vi "UHR-Fleezers Control (host) - 10.2.vi"() -> ()   [LabVIEW 2009] (continued)
  out "All Signals":waveform(dbl)[](graph)=[{"t0"=timestamp(9589.800000000116 s since 1904-01-01), "dt"=0.15, "Y"=[380.0, 400.0], "attributes"=variant("NI_ChannelName"=variant(string "APD 1"))}, {"t0"=timestamp(9589.800000000116 s since 1904-01-01), "dt"=0.15, "Y"=[140.0, 160.0], "attributes"=variant("NI_ChannelName"=variant(string "APD 2"))}, {"t0"=timestamp(9589.800000000116 s since 1904-01-01), "dt"=0.15, "Y"=[-0.5560947071135384, -0.5488051268739088], "attributes"=variant("NI_ChannelName"=variant(string "T1 Y"))}, {"t0"=timestamp(9589.800000000116 s since 1904-01-01), "dt"=0.15, "Y"=[-0.6964523017525798, -0.7003016638635213], "attributes"=variant("NI_ChannelName"=variant(string "T1 X"))}, {"t0"=timestamp(9589.800000000116 s since 1904-01-01), "dt"=0.15, "Y"=[0.009100131229590747, 0.009068117313150425], "attributes"=variant("NI_ChannelName"=variant(string "T1 Sum"))}, {"t0"=timestamp(9589.800000000116 s since 1904-01-01), "dt"=0.15, "Y"=[-0.557341526703397, -0.5498308802934172], "attributes"=variant("NI_ChannelName"=variant(string "T2 Y"))}, {"t0"=timestamp(9589.800000000116 s since 1904-01-01), "dt"=0.15, "Y"=[-0.6977537048097585, -0.7016458986193993], "attributes"=variant("NI_ChannelName"=variant(string "T2 X"))}, {"t0"=timestamp(9589.800000000116 s since 1904-01-01), "dt"=0.15, "Y"=[0.009161107211523788, 0.00913434247871334], "attributes"=variant("NI_ChannelName"=variant(string "T2 Sum"))}, {"t0"=timestamp(9589.800000000116 s since 1904-01-01), "dt"=0.15, "Y"=[0.05199389581726632, 0.0511983167557167], "attributes"=variant("NI_ChannelName"=variant(string "T1 FB X"))}, {"t0"=timestamp(9589.800000000116 s since 1904-01-01), "dt"=0.15, "Y"=[0.016877803888058106, 0.01688229010895108], "attributes"=variant("NI_ChannelName"=variant(string "T1 FB Sum"))}, {"t0"=timestamp(9589.800000000116 s since 1904-01-01), "dt"=0.15, "Y"=[0.048074905987419425, 0.04747925277569201], "attributes"=variant("NI_ChannelName"=variant(string "T2 FB X"))}, {"t0"=timestamp(9589.800000000116 s since 1904-01-01), "dt"=0.15, "Y"=[0.016815240943632313, 0.016807855464339123], "attributes"=variant("NI_ChannelName"=variant(string "T2 FB Sum"))}, {"t0"=timestamp(9589.800000000116 s since 1904-01-01), "dt"=0.15, "Y"=[-3.8792427407756658, -3.877178718972479], "attributes"=variant("NI_ChannelName"=variant(string "PSD Y"))}, {"t0"=timestamp(9589.800000000116 s since 1904-01-01), "dt"=0.15, "Y"=[-0.32047881103365267, -0.32100188649167594], "attributes"=variant("NI_ChannelName"=variant(string "PSD X"))}, {"t0"=timestamp(9589.800000000116 s since 1904-01-01), "dt"=0.15, "Y"=[-0.025290139469588305, -0.02530741294595172], "attributes"=variant("NI_ChannelName"=variant(string "PSD Y Sum"))}]
  in  "Signals to Plot":i32(listbox)
  out "Trap Disp. Freq. (Hz)":dbl=6.666666666666667 caption="Freq. (Hz)" format="%#_6p"
  out "Display Period (s)":dbl=0.15 caption="Period (s)" format="%#_6p"
  in  "Trap Disp. Downsample":dbl=10000.0 caption="Downsample" max=20000.0
  in  "APD Disp. Scale":dbl=0.1 caption="Scale (Divide,\nfor above plot only)"
  in  "APD Disp. Downsample":dbl=15.0 caption="Integrate" min=1.0 max=30.0 step=1.0
  out "APD Display Freq. (Hz)":dbl=6.666666666666667 caption="Freq. (Hz)"
  out "APD Display Period (s)":dbl=0.15 caption="Period (s)"
  out "FFT 1":cluster{"f0":dbl, "df":dbl, "magnitude":dbl[]}[](graph)=[{"f0"=0.0, "df"=3.3333333333333335, "magnitude"=array[10000 elements]}, {"f0"=0.0, "df"=3.3333333333333335, "magnitude"=array[10000 elements]}]
  out "FFT 2":cluster{"f0":dbl, "df":dbl, "magnitude":dbl[]}[](graph)
  in  "FFT 1 Choice 1":u16(ring) items=["T1 Y", "T1 X", "T1 Sum", "T2 Y", "T2 X", "T2 Sum", "T1 FB X", "T1 FB Sum", "T2 FB X", "T2 FB Sum", "PSD Y", "PSD X", "PSD Y Sum", "none"]
  in  "FFT 2 Choice 1":u16(ring)=13 items=["T1 Y", "T1 X", "T1 Sum", "T2 Y", "T2 X", "T2 Sum", "T1 FB X", "T1 FB Sum", "T2 FB X", "T2 FB Sum", "PSD Y", "PSD X", "PSD Y Sum", "none"]
  in  "FFT 1 Choice 2":u16(ring)=1 items=["T1 Y", "T1 X", "T1 Sum", "T2 Y", "T2 X", "T2 Sum", "T1 FB X", "T1 FB Sum", "T2 FB X", "T2 FB Sum", "PSD Y", "PSD X", "PSD Y Sum", "none"]
  in  "FFT 2 Choice 2":u16(ring)=13 items=["T1 Y", "T1 X", "T1 Sum", "T2 Y", "T2 X", "T2 Sum", "T1 FB X", "T1 FB Sum", "T2 FB X", "T2 FB Sum", "PSD Y", "PSD X", "PSD Y Sum", "none"]
  in  "Compute FFT":bool
  in  "Reset FFT":bool
  in  "# Spectra to Ave.":dbl=25.0
  out "Ave. Time (s)":dbl=7.5
  out "1 Channel":waveform(dbl)(graph)={"t0"=timestamp(0 s since 1904-01-01), "dt"=1.4999999999999999e-05, "Y"=array[20000 elements], "attributes"=variant("NI_ChannelName"=variant(string "T1 Y"))}
  out "Slow mean":dbl=0.04741485510254009 format="%0.2f"
  in  "Slow mean N ave.":dbl=1.0 min=1.0 step=1.0
  out "Mean Intensity":dbl=0.04741485510254009
  out "Sigma":dbl=0.006116447585273888
  out "Sigma/Mean":dbl=0.12899855060289364
  in  "Subtract mean":bool
  in  "High Res. Display":u16(ring) items=["T1 Y", "T1 X", "T1 Sum", "T2 Y", "T2 X", "T2 Sum", "T1 FB X", "T1 FB Sum", "T2 FB X", "T2 FB Sum", "PSD Y", "PSD X", "PSD Y Sum"]
  out "APD 1 Rate (Hz)":dbl=330.0 format="%#_3p"
  in  "Tab Control":T4(tab)=enum."APD Counting"
  out "Stage Moving":bool
  in  "Read Cal":bool
  in  "Confocal Linescan":bool
  in  "Speed (nm/s)":dbl=100.0
  in  "Furthest Withdraw (MHz)":dbl=15.0
  in  "Confocal Image":bool
  in  "Round T1 X":bool caption="Round"
  in  "T1 offset_x (mV)":dbl=-63.86439785165793 format="%#_2g"
  in  "T1 kappa_x (pN/nm)":dbl=0.25444062839906995 min=0.0 step=0.001 format="%#_2g"
  out "Time (s)":dbl=8.7
  out "Total Time (s)":dbl=60.0
  in  "Start Saving":bool
  in  "Cal sets to save":u32=50 min=1 step=1
  in  "Comment (data description)":string="testing confocal setup"
  out "Calibrating Trap...":bool
  in  "Trap 2 (ON/OFF)":bool
  in  "Trap 1 (ON/OFF)":bool
  in  "Save Calibration":bool
  in  "N sets to save":u32=200 caption="N Sets"
  in  "Save N Sets":bool
  out "Save file name":path=path "E:/Data/101209/101209_067.dat"
  in  "Save ave N":dbl=500.0 caption="Averaging Factor"
  out "Saving...":bool
  in  "Stop Saving":bool
  out "Progress":u16(slide) scale=0.0..100.0
  out "Manipulating Trap":bool
  out "Buffer Status":dbl(slide) scale=0.0..1.0
  out "Overflow (data lost)":bool
  in  "Reset":bool
  out "Data Rate (Hz)":dbl=66666.66666666667 caption="Trap Data Rate (Hz)" format="%#_3p"
  out "Data Period (s)":dbl=1.4999999999999999e-05 caption="Trap Data Period (s)" format="%#_6p"
  out "Save Data Rate (Hz)":dbl=133.33333333333334 caption="Rate (Hz)" format="%#_6p"
  out "Save Data Period (s)":dbl=0.0075 caption="Period (s)" format="%#_6p"
  in  "T1 alpha_x (nm/V)":dbl=668.456221254379 step=10.0 format="%#_3g"
  in  "T2 alpha_x (nm/V)":dbl=772.4433031277968 step=10.0 format="%#_3g"
  in  "T2 kappa_x (pN/nm)":dbl=0.21976131273941338 min=0.0 step=0.001 format="%#_2g"
  in  "T2 offset_x (mV)":dbl=-64.70019248344109 format="%#_2g"
  in  "BD 1 Frequency 1 (MHz)":dbl=72.0 caption="T1 X (MHz)" min=60.0 max=90.0 step=1.0 format="%#_6p"
  in  "BD 1 Frequency 2 (MHz)":dbl=85.0 caption="T2 X (MHz)" min=60.0 max=90.0 step=1.0 format="%#_6p"
  in  "Green Laser ON/Interlacing":bool
  in  "Round T2 X":bool caption="Round"
  in  "AO1":dbl(slide)=5.724448901115672 caption="Confocal Y (V)" min=0.0 max=10.0 step=0.01 scale=0.0..10.0 scale format="%_1f"
  in  "AO2":dbl(slide)=2.676722922452468 caption="Confocal X (V)" min=0.0 max=10.0 step=0.01 scale=0.0..10.0 scale format="%_1f"
  in  "Trap Raster Scan":bool
  out "Raster Scanning...":bool
  in  "Trap Delta (MHz)":dbl=13.0
  in  "Setpoints (V)":cluster{"Set 1":dbl, "Set 2":dbl}={"Set 1"=9.0, "Set 2"=9.0}
  in  "Index":dbl=67.0 caption="Save File Index" min=1.0 step=1.0
  in  "Position Label 5":string="upper flow spot (UvrD)" caption="5"
  in  "Move to Position":bool
  in  "Position":dbl=1.0 min=1.0 max=10.0 step=1.0
  in  "Set Position":bool
  in  "Saved Stage Positions":dbl[][](array[numeric])=[[1.0, 1.95922, -0.44604, 0.0063], [2.0, 0.0, 0.0, 0.0], [3.0, 2.85199, -0.5102, 0.0063], [4.0, -0.33267, -0.41387, -0.00044], [5.0, 2.804, -1.87124, -0.00044], [6.0, 0.0, 0.0, 0.0], [7.0, 0.0, 0.0, 0.0], [8.0, 0.0, 0.0, 0.0], [9.0, 0.0, 0.0, 0.0], [10.0, 0.0, 0.0, 0.0]]
  in  "Move to Position 5":bool
  in  "z nudge increment (um)":dbl=0.5
  in  "+z":bool
  in  "Position 1 Label":string="Right capillary (DNA beads)" caption="1"
  in  "Set Position 1":bool
  in  "Set Position 2":bool
  in  "Set Position 3":bool
  in  "Set Position 4":bool
  in  "Move to Position 3":bool
  in  "Move to Position 4":bool
  in  "Move to Position 2":bool
  in  "Move to Position 1":bool
  in  "Position 2 Label":string="Left capillary (ADig beads)" caption="2"
  in  "Position 3 Label":string="lower flow spot (ATP)" caption="3"
  in  "Position 4 Label":string="Dump beads" caption="4"
  in  "-z":bool
  in  "Set Position 5":bool
  out "Stage Control Serial Error":errorcluster={"status"=FALSE, "code"=1073676293, "source"="VISA Read in Set Stage Position.vi->UHR-Fleezers Control (host) - 10.2.vi"}
  out "Pump 3 cont disp":string="Left: ADig beads"
  out "Pump 1 cont disp":string="Right: DNA beads "
  in  "Ch 1 Inject Rate (ul/h)":dbl=100.0
  in  "Pump write delay (ms)":dbl=300.0
  in  "All Pump Parameters":T5={"Pump 1"={"Diameter (mm)"=4.61, "Units"=4.0, "Volume"=100.0, "Rate"=100.0}, "Pump 2"={"Diameter (mm)"=4.61, "Units"=3.0, "Volume"=0.0, "Rate"=0.0}, "Pump 3"={"Diameter (mm)"=4.61, "Units"=4.0, "Volume"=100.0, "Rate"=200.0}}
  in  "Ch 2 Inject Volume (uL)":dbl=100.0
  in  "Pump pause delay (ms)":u32
  in  "Ch 3 Inject Volume (uL)":dbl=100.0
  in  "Ch 3 Inject Rate (ul/h)":dbl=200.0
  in  "Flush Center Ch Volume (uL)":dbl=15.0
  in  "Flush Center Ch Rate (ul/m)":dbl=100.0
  in  "Inject Pump 2":bool caption="Inject Pump 2\n(Flush Center)"
  in  "Total Volume\nFlushed (uL)":dbl
  in  "Tab Control 2":T6(tab)=enum."Feedback on Trap Position"
  out "Total Counts (ticks)":u32=600
  in  "Trap ON/OFF X or Y Amp?":bool=TRUE
  in  "Oscillate Set 1":bool
  in  "Trap 1 ON":bool
  in  "Number Interlace Sets":u8=3 min=1 max=3
  in  "DIO count 3 (ticks)":u32=200
  in  "DIO count 2 (ticks)":u32=200
  in  "DIO count 1 (ticks)":u32=200
  in  "BD 2 Amplitude 3 (%)":dbl min=0.0 max=50.0 step=1.0
  in  "BD 2 Amplitude 2 (%)":dbl min=0.0 max=50.0 step=1.0
  in  "BD 2 Amplitude 1 (%)":dbl min=0.0 max=50.0 step=1.0
  in  "BD 1 Amplitude 3 (%)":dbl min=0.0 max=50.0 step=1.0
  in  "BD 1 Amplitude 2 (%)":dbl=35.0 min=0.0 max=50.0 step=1.0
  in  "BD 1 Amplitude 1 (%)":dbl=10.0 min=0.0 max=50.0 step=1.0
  in  "BD 2 Frequency 3 (MHz)":dbl=26.0 min=0.0 max=40.0 step=1.0 format="%#_6p"
  in  "BD 1 Frequency 3 (MHz)":dbl=70.0 min=60.0 max=90.0 step=1.0 format="%#_6p"
  in  "BD 2 Frequency 2 (MHz)":dbl=26.0 min=0.0 max=40.0 step=1.0 format="%#_6p"
  in  "BD 2 Frequency 1 (MHz)":dbl=26.0 min=0.0 max=40.0 step=1.0 format="%#_6p"
  in  "Not-Interlacing Set":enum32{"Set 1", "Set 2", "Set 3"}(radio)
  in  "Interlace":bool=TRUE
  in  "Trap 2 ON":bool
  in  "Trap 3 ON":bool
  in  "Scan axis 2":bool=TRUE
  in  "Osc. freq. (Hz)":dbl=0.25
  in  "Osc. amp. (MHz)":dbl=2.0
  out "Coords":T7
  in  "Manipulation Scaling":cluster{"Horizontal":dbl, "Vertical":dbl}={"Horizontal"=0.075, "Vertical"=0.01}
  in  "Freq or Amp switch first":bool=TRUE
  in  "Swap F1 and F2":bool
  in  "Freq switch delay":u16
  in  "Amp switch delay":u16=5
  in  "MCL Step Increment (V_int)":dbl=3.0
  out "Time to Finish All (min)":dbl=0.13986 format="%#_2p"
  in  "Scan Speed (nm/s)":dbl=100.0
  in  "Scan Range (nm)":dbl=420.0
  in  "Step Size (nm)":dbl=1.0
  in  "MCL/AOM Scale Tweak":dbl=1.0
  in  "MCL Step Position Ratio":dbl=0.5
  in  "Move MCL Also?":bool=TRUE
  out "Final sep (nm)":dbl=1194.000000000001
  out "Initial sep (nm)":dbl=774.0
  out "Save index":dbl=67.0
  out "Final delta (MHz)":dbl=16.41463414634147
  out "Initial delta (MHz)":dbl=13.0
  out "Final freq. (MHz)":dbl=68.58536585365853
  out "Initial freq. (MHz)":dbl=72.0
  in  "Saved AOD Raster Scan Parameter Sets":T8(array[cluster])=[{"Scan Range AOD (nm) 2"=500.0, "Step Size AOD (nm) 2"=1.0, "Scan Speed AOD (nm/s) 2"=100.0, "Number of scans (AOD) 2"=1, "Label"="offset curve"}, {"Scan Range AOD (nm) 2"=420.0, "Step Size AOD (nm) 2"=1.0, "Scan Speed AOD (nm/s) 2"=100.0, "Number of scans (AOD) 2"=1, "Label"="hp raster check"}, {"Scan Range AOD (nm) 2"=6.8, "Step Size AOD (nm) 2"=0.34, "Scan Speed AOD (nm/s) 2"=0.34, "Number of scans (AOD) 2"=1, "Label"="3.4 kbp - 1 bp steps"}]
  in  "Load parameters":bool
  out "Scan Range (MHz)":dbl=-3.4146341463414633
  in  "Restart DMA? (AOD)":bool=TRUE caption="Restart DMA?"
  out "Incr. int (AOD)":i64=-7759651845
  out "Time/Scan (s) (AOD)":dbl=4.1958 format="%#_2p"
  out "Data points/scans":dbl=559440.0
  out "Data points/scan (f/b)":dbl=559440.0
  in  "Save scans":bool=TRUE
  out "AOD Scan I":u64=2 caption="Scan I"
  in  "Continuous AOD Scanning":bool caption="Continuous Scanning"
  in  "Abort AOD Scan":bool caption="Abort Scan"
  in  "Scan BD":bool=TRUE
  out "Cycles/step (AOD)":u64=666 format="%.3p"
  in  "Number of F/B Scans (AOD)":u16=1 min=1
  out "Scan steps (AOD)":u64=420
  out "Scan Increment (MHz)":dbl=-0.008149484836137144
  out "AOD Scanning":bool caption="Scanning"
  in  "Start AOD Scan":bool caption="Start Scan"
  out "N sets should be saved":dbl=27.972
  out "Progress 2":u16(slide) caption="Progress" scale=0.0..100.0
  in  "Abort save 2":bool caption="Abort save"
  in  "Trap 1 Bead Size (nm)":dbl=860.0
  in  "Trap 2 Bead Size (nm)":dbl=790.0
  out "MCL Count":dbl=782931.6080202643
  in  "All FB On/Off":bool=TRUE
  in  "AI2 to Setpoint":cluster{"Set 1":bool, "Set 2":bool}
  out "AI2 (V)":cluster{"Set 1":dbl, "Set 2":dbl}={"Set 1"=0.017090365306558428, "Set 2"=0.016785180211798457}
  in  "Reset Feedback":cluster{"Set 1":bool, "Set 2":bool}
  in  "PID Gains":T9={"Set 1"={"proportional gain (Kc)"=0, "integral gain (Kc*Ts/Ti)"=5, "derivative gain (Kc*Td/Ts)"=0}, "Set 2"={"proportional gain (Kc)"=0, "integral gain (Kc*Ts/Ti)"=5, "derivative gain (Kc*Td/Ts)"=0}}
  in  "Feedback On/Off":cluster{"Set 1":bool, "Set 2":bool}={"Set 1"=TRUE, "Set 2"=TRUE}
  in  "Set SP to Reading":bool
  out "Trap X (AI1)":T10={"Trap 1"=-0.375, "Trap 2"=-0.381805419921875}
  in  "Trap Pos FB SP":fxp<+/-,16,1>=-0.123443603515625 caption="Setpoint"
  in  "Trap Pos. FB ON":bool
  in  "Reset Trap Pos. FB":bool
  out "Trap Positions":waveform(dbl)[](graph)=[{"t0"=timestamp(9589.800000000116 s since 1904-01-01), "dt"=0.15, "Y"=[0.0, 0.0], "attributes"=variant("NI_ChannelName"=variant(string "Trap 1 Pos."))}, {"t0"=timestamp(9589.800000000116 s since 1904-01-01), "dt"=0.15, "Y"=[5.5933924159035087e-11, 5.5933924159035087e-11], "attributes"=variant("NI_ChannelName"=variant(string "Trap 2 Pos."))}]
  in  "Tab Control 8":enum32{"Main Setting", "Details"}(tab)=enum."Details"
  in  "Trap Pos FB Int Count":u16=100
  in  "Trap Pos. FB Gains":T11={"proportional gain (Kc)"=10.0, "integral gain (Kc*Ts/Ti)"=10.0, "derivative gain (Kc*Td/Ts)"=0.0} {"proportional gain (Kc)" format="%.11g"; "integral gain (Kc*Ts/Ti)" format="%.11g"; "derivative gain (Kc*Td/Ts)" format="%.11g"}
  in  "Trap Pos. FB Offset Factor":i64
  in  "Trap Pos FB Negate Action":bool
  in  "Trap Pos. FB Mult Factor":i64=8388608
  in  "Trap Pos. AI1 X Pre-scale":u16
  in  "Trap Pos. FB Range":T12={"output high"=0.999969482421875, "output low"=-1.0}
  out "Trap Pos FB Int Signal":fxp<+/-,24,9>=-5.86773681640625 format="%.18g"
  out "Trap Pos FB Int-Norm Signal":fxp<+/-,16,1>=-0.058685302734375 format="%.16g"
  in  "Set SP Using...":bool
  in  "Trap Pos FB Monitor\nT1 or T2":bool
  out "Trap X AI1 (DMA)":T13={"Set 1"=-0.700286865234375, "Set 2"=-0.70166015625}
  in  "N El. to Ave.":dbl=10000.0
  out "Trap Pos FB Action":i64=-32768
  out "Action (%)":dbl(knob)=-100.0030518509476 scale=-100.0..100.0
  in  "Trap Pos. FB Out Scale 2^n":u8=23 caption="Action Scale"
  out "Mean T1 Position (nm)":dbl caption="Mean T1 (nm)" format="%0.2f"
  out "Trap 1 Position RMS (A)":dbl caption="RMS (Ang)"
  in  "Tab Control 3":enum32{"Timing", "MCL Scan", "Analog Out"}(tab)
  in  "On one out of X cycles":dbl=1.0
  out "APD 2 Gate Late Counter":u32
  out "APD 2 Gate Relative Phase":i16
  in  "Phase Adj. (APD 2 Gate)":i16=20
  in  "Initial Phase Adjustment (APD 2 Gate)":i16=55
  out "APD 1 Gate Late Counter":u32
  in  "- phase (APD 1 Gate)":bool
  in  "+ phase (APD 1 Gate)":bool
  out "APD 1 Gate Relative Phase":i16
  in  "Phase Adj. (APD 1 Gate)":i16=20
  in  "Initial Phase Adjustment (APD 1 Gate)":i16=60
  in  "Save APD Data\nwith Trap Data":bool=TRUE
  out "APD FIFO Elements Remaining":u32
  in  "- phase (APD Acq)":bool
  in  "+ phase (APD Acq)":bool
  out "APD Acq Late Counter":u32
  out "APD Acq Relative Phase":i16
  in  "Phase Adj. (APD Acq)":i16=20
  in  "Initial Phase Adjustment (APD Acq)":i16
  in  "Invert APD Gate":bool caption="Invert Gate"
  in  "APD Gate OFF Count":u32=450 caption="Gate OFF Count"
  in  "APD Gate ON Count":u32=150 caption="Gate ON Count"
  in  "APD Gate":enum32{"ON", "OFF", "Interlace"}(radio)=enum."Interlace"
  in  "APD Integration Time (s)":dbl=0.01 caption="Integration Time (s)"
  out "APD Acq Rate (Hz)":dbl=100.0 caption="Rate (Hz)"
  out "APD Samples/FIFO Acq.":dbl=30.0
  out "APD Elements/DMA read":u32=60
  out "APD Int. Count":u32=400000 format="%.0p"
  in  "+ phase (APD 2 Gate)":bool
  in  "- phase (APD 2 Gate)":bool
  in  "Tab Control 5":enum32{"PSD X", "PSD Y", "Other Data Channel"}(tab)
  out "Data map":dbl[][](graph)=[[-0.1333528275848164, -0.13322457942865132, -0.13338141499330441, -0.13315516332872823, -0.13349963906401516, -0.13359534704399442, -0.1336383102533325, -0.1334437596814232, -0.13351009901028432, -0.133174726924376, -0.13353618610342308, -0.13341430673495425, -0.1337791921327295, -0.13336672306878955, -0.13358485673285964, -0.13386556704797015, -0.13364109162411741, -0.1331515440816014, -0.13347705703506113, -0.13332438096152477], [-0.13330982878455255, -0.1332750495144987, -0.13319436165006812, -0.13320436012398332, -0.13337780682419856, -0.13318346406303316, -0.13354384273485564, -0.1335553857723867, -0.1333855860720205, -0.13344880369084505, -0.13331726120488946, -0.13359903256786615, -0.13374990418036614, -0.13320003077320358, -0.13320258284496916, -0.13349625923097894, -0.13341762191515427, -0.13321738360286317, -0.13365332165632604, -0.13336876386087104], [-0.13338432873053255, -0.13369836704787957, -0.13302853528383926, -0.13284664713529393, -0.13331163931728274, -0.1333869240906723, -0.1333441110818246, -0.13363613855507872, -0.13328973057954627, -0.13338978606911753, -0.13344572107757746, -0.1335788632456775, -0.13369207672074693, -0.1333552666645917, -0.133366088161167, -0.13353851024718505, -0.13344522029848654, -0.13326189706976171, -0.13331998061539002, -0.1334005748287191], [-0.133325559644922, -0.13328193405696326, -0.13298363395722104, -0.1327420972940746, -0.13319836061291315, -0.13335561564627363, -0.13332406410277234, -0.1332193936628136, -0.133421455482787, -0.13322247098645962, -0.1334396039903118, -0.13383402308145578, -0.13367469216535152, -0.13342428864571734, -0.13322726574810206, -0.13374616438110215, -0.13359839386433672, -0.13308981369306616, -0.13346933931556157, -0.13356004700673044], [-0.13318759427178156, -0.13303197461884955, -0.1329474628909061, -0.13247541089967585, -0.1329154393010578, -0.13306639647153298, -0.13294170402663102, -0.13330832394952757, -0.13324788676517313, -0.13321368995590022, -0.1332902540311242, -0.13330558882916305, -0.13358290232698766, -0.13297453395748215, -0.13345940796964523, -0.13370893335312267, -0.13345621914098815, -0.1329981434590732, -0.13351225698035923, -0.13366090449522447], [-0.1330195631246013, -0.1332342730086348, -0.13270649932352258, -0.13215920438073567, -0.13266516267281567, -0.13295697773848095, -0.13293578982905166, -0.13287245269750408, -0.13242956314631302, -0.13269915277373706, -0.13276507119029501, -0.1330605974520571, -0.13298007789861815, -0.13297345004496647, -0.13322005694115485, -0.13306352360169843, -0.13330195770575692, -0.13273863763579463, -0.13328311983926244, -0.1334693235390487], [-0.13266227273000536, -0.13265909726526673, -0.13248512915752836, -0.13206858076806094, -0.13237793289780897, -0.13264412379816848, -0.13258756757327542, -0.1320114058200433, -0.13177271172238408, -0.131641684580745, -0.1313885201234832, -0.13157327086959134, -0.13193681668173818, -0.13205110975662787, -0.13214611067498203, -0.1325055082405619, -0.13286551272419084, -0.1327044073944107, -0.13314434714805756, -0.13328319140887135], [-0.1322287995794756, -0.13244081796536053, -0.1320813927793243, -0.13167992350139204, -0.13159036903481355, -0.1309389927960272, -0.13012719192929267, -0.12950031847514665, -0.1287847279946542, -0.12849799334601392, -0.12875851379831316, -0.1291683370175165, -0.12945041921408823, -0.13011135722738026, -0.13068229553908456, -0.13178041385585593, -0.13210874887914992, -0.13240101800950432, -0.13307651459147396, -0.1332815698201827], [-0.13168864185361212, -0.13169057747645646, -0.13094174949231982, -0.1296062475621515, -0.12911771760332813, -0.1277654225075574, -0.12620502956235657, -0.12542678436739468, -0.12488401076433495, -0.12466156919740522, -0.12464721211960658, -0.12569461568122886, -0.12655494067992784, -0.12794364582857165, -0.12901026270421723, -0.13041242181451723, -0.1309906967933238, -0.13192115434221466, -0.13278733750759975, -0.13294457795155415], [-0.13140698916298538, -0.13053117104461706, -0.1298789379990306, -0.12819663899680442, -0.12676039208733167, -0.12543956236126258, -0.12399151681160528, -0.12321545134257084, -0.12266144922386354, -0.12308476056426831, -0.12333356428193396, -0.12442839177134496, -0.125361994472599, -0.1263601593064314, -0.12820727599853887, -0.1295078859250952, -0.13070166715851583, -0.13132458320754442, -0.13239984696061652, -0.13272823213845275], [-0.1316630563769322, -0.13058177067274154, -0.12934738039745952, -0.1279160589030836, -0.12698760416503796, -0.1261278846897266, -0.12563290805554983, -0.12525048180917475, -0.12499775033256465, -0.12548503096818717, -0.12562927805994936, -0.12652509628180203, -0.1268728117841831, -0.12754090298678572, -0.128892648954199, -0.1303663985392085, -0.13107103289262145, -0.13211332838117568, -0.13253399544795413, -0.13320687544530033], [-0.13216081866528823, -0.1315075999575009, -0.13100587070574482, -0.12992811693100018, -0.12997653166936626, -0.1292147140061146, -0.129640492236645, -0.12897956592947535, -0.12976715583017567, -0.1297932787035981, -0.1298023450792772, -0.13032188725883695, -0.1304761361878746, -0.13078161341726655, -0.13166629776722513, -0.13222471508906133, -0.1323213695353957, -0.1328207574902124, -0.13311501551624966, -0.1332632433913324], [-0.13281254318355107, -0.1327562901435425, -0.1326441296540774, -0.13233527591102084, -0.13266449238724481, -0.13265305237392538, -0.1332895530560203, -0.1328797037513923, -0.1337875611075738, -0.1338856032262169, -0.13396272235535894, -0.13467820635255304, -0.13459472658495253, -0.13481512721792738, -0.13510227952708725, -0.13479149504020294, -0.1342173989040399, -0.13400692912651818, -0.13384849198616516, -0.13400637529892312], [-0.13375357959243867, -0.13404569542560457, -0.13495364446143102, -0.1348249298919473, -0.13511113811042258, -0.13586064734534106, -0.1367702427345483, -0.13640277389675376, -0.137350097056054, -0.13768947654536537, -0.1377600167625419, -0.13864975659183087, -0.13855745695114235, -0.13847369645672247, -0.13797396835814926, -0.13685971442597938, -0.13588001721479026, -0.1348828617294378, -0.13459338431719314, -0.13430841037731373], [-0.13472163516252944, -0.13510778933514528, -0.13606324391762598, -0.13721477688556563, -0.13796918063942398, -0.13907970504607353, -0.13997063223219003, -0.1404952519216667, -0.14116015514376445, -0.14184210813677695, -0.14195006345681294, -0.1422200144829778, -0.14146161292344456, -0.14066503891408247, -0.13917249864709688, -0.13787213188733544, -0.13644632375244403, -0.13531181544046453, -0.13475242805372128, -0.13409655719999836], [-0.1346275621787114, -0.13581997744258686, -0.13673753910551079, -0.13825764083372993, -0.1393970856121808, -0.14055132722262284, -0.14212435341131746, -0.1429946497851761, -0.14389674915902945, -0.14437685341315143, -0.14394884392741297, -0.1437461923774046, -0.14212089804047442, -0.14062257694636499, -0.1389648070082139, -0.13735907714557666, -0.13619045970534122, -0.13491396011330425, -0.13433155550518988, -0.13385926149247016], [-0.1345463015984732, -0.13533049006777814, -0.1360079415666268, -0.13724519284297043, -0.13796266414019026, -0.13972197426375965, -0.140812875728494, -0.14160716758492864, -0.14245424606827867, -0.1426660914472218, -0.1419273669362709, -0.1411193505685126, -0.1396820763279355, -0.13849550538403904, -0.1371160534173631, -0.13616108727356172, -0.1350846968502612, -0.1345579784231545, -0.13422057092103412, -0.13391963188088524], [-0.1345140812644617, -0.13453873857919768, -0.13492439205985124, -0.13522924105885664, -0.13553263780450764, -0.13682685486563656, -0.13746523593705381, -0.13769959429766693, -0.13823681534599064, -0.13804540570103968, -0.1377168473234902, -0.137249678692798, -0.13663158321787355, -0.1358724287761378, -0.13508757455503823, -0.13481824547523152, -0.13451280366787882, -0.13405512825859384, -0.13357356099604073, -0.13361557829424386], [-0.13375329911523637, -0.1339884743615168, -0.13405049775855704, -0.13387302958751493, -0.13446815488578315, -0.13456307392704003, -0.1348368701021389, -0.1346671744649869, -0.1351616786066821, -0.13494184842817455, -0.13482617852864523, -0.13488001595602087, -0.13479250678601862, -0.13422794469954447, -0.13407231195254116, -0.13428834815292778, -0.13391074942860734, -0.1335842092801955, -0.13360705080299462, -0.13369073131918308], [-0.13342007903772915, -0.13363428924338872, -0.1336865137711592, -0.13362267437830241, -0.1340879064681812, -0.1343702460433723, -0.13427212990252296, -0.13438113623254638, -0.1342984197115018, -0.13454000136156902, -0.13410240023843895, -0.13431191302358195, -0.13372696338190082, -0.13351446601080696, -0.13369323044331194, -0.13382214512554041, -0.1335590429270594, -0.13334703606343876, -0.13344861559376253, -0.13363740432965837], [-0.13345101950898047, -0.13370694960200571, -0.13375272427901636, -0.13367615478109512, -0.133581419993757, -0.13404024017347133, -0.13403381313279544, -0.13412766960211026, -0.13408917169871215, -0.1340991529228964, -0.13394020765617004, -0.13411866463837074, -0.1338152058493298, -0.1334965001552756, -0.1336131483128123, -0.13359828229506895, -0.13336465129415692, -0.13314738412311986, -0.13348416355472054, -0.1335604277916293], [-0.13306505037644084, -0.13323849362189907, -0.13358463035347495, -0.13325024737032973, -0.1339034907224333, -0.1334823513422517, -0.13364118194855779, -0.13370487605571307, -0.13388403686022388, -0.13370936861025146, -0.13365536795624064, -0.13368173604417122, -0.13323022669565254, -0.1334299644310924, -0.13347931020293585, -0.13352842249169267, -0.13337684428363186, -0.13325924288621083, -0.13329745168878554, -0.1337439591709793], [-0.13329253323559506, -0.1331777915331699, -0.1335921549944053, -0.1328937870573285, -0.1332366580681567, -0.13343263834499086, -0.1334011301059611, -0.1333309838285126, -0.13350159936016623, -0.13320469976499644, -0.13344779732284073, -0.1334547498891746, -0.1334222219690806, -0.13318482310735769, -0.1335076304440751, -0.1337210081454326, -0.13315452452181906, -0.1334159900117032, -0.13341932871289236, -0.13354841337059192], [-0.13280291955733525, -0.13325064759222977, -0.13311404335060162, -0.13248463689492918, -0.1333237715792868, -0.1323786195149216, -0.13271644461940252, -0.13281630630206784, -0.13288259797605967, -0.13249986045502704, -0.13281665454186062, -0.13272056012529576, -0.13286471860468907, -0.13278402529871713, -0.13291014412980584, -0.13297993805663647, -0.13300434625587784, -0.1330929771016705, -0.13330992360244986, -0.13370648866336798], [-0.13245142727010079, -0.1327511055284677, -0.13268045863644556, -0.13268143112611724, -0.1325461389457877, -0.13209427203867338, -0.1321009552727226, -0.13225536226981105, -0.13186019651868192, -0.13057556692968597, -0.13114921940462385, -0.1309652877414555, -0.13152741909874535, -0.1317933488461379, -0.13157278355428226, -0.1320550574560594, -0.13258159805880432, -0.1325290720118073, -0.1330325946278319, -0.13335799111764524], [-0.132440641977841, -0.13223274943079838, -0.13289269966476258, -0.13166651817936692, -0.13145823100189755, -0.13071613425469086, -0.1305561586856538, -0.1298730961500496, -0.12931009768505008, -0.1282939344060649, -0.12877776236794292, -0.12861422530652827, -0.12939444719778675, -0.12959820237747077, -0.12982084600249316, -0.13091293127431075, -0.13161604230879553, -0.13196152998858568, -0.13235636411870588, -0.13286676513248602], [-0.1320090784600222, -0.1320251702775283, -0.1320201366202131, -0.1308841791296303, -0.13024919149293854, -0.12882972626185074, -0.12841801068211917, -0.1277257404207089, -0.12729636083194423, -0.12612102323152535, -0.1266176500993184, -0.12699800464045685, -0.1273436224975044, -0.12801691442078328, -0.1285301864636645, -0.12982378997391497, -0.13037226121792483, -0.1309877220002564, -0.13195835248531285, -0.1327283377905438], [-0.13219445798910656, -0.13188688269527568, -0.1312592281486657, -0.12974550875405527, -0.12950618274953632, -0.1282777123290045, -0.12815500917958844, -0.1276867543572287, -0.12753413346428072, -0.12700805569043083, -0.12731245292472204, -0.12733022642180977, -0.12794125592111183, -0.12787103039057496, -0.12851092699043953, -0.12941433262690494, -0.1302167567007781, -0.13097544099877062, -0.1313019129364665, -0.13256884384406073], [-0.13203935721135476, -0.1319797555557467, -0.13125504649143416, -0.1306737121404095, -0.13023153377695054, -0.12962817928808207, -0.12967599795049806, -0.12935147357664667, -0.12930920917934416, -0.12932450565660736, -0.12960389680547735, -0.12972037405457418, -0.1297802847172711, -0.12990558188238963, -0.12998660414360977, -0.13060943118902887, -0.1309291374525452, -0.13126102756068508, -0.1317875372713273, -0.13289602021495517], [-0.13237209389326543, -0.13252267873479864, -0.1322605318662779, -0.13185876549480874, -0.13161073280800273, -0.1316314093234348, -0.13175685738586845, -0.1316715289616997, -0.13176387169644788, -0.13178347463822943, -0.13222097937928162, -0.13203755361500033, -0.13189928703016512, -0.13207046955652132, -0.13193239985056698, -0.13238530821059563, -0.13213549192663696, -0.13225053431681083, -0.13249723798670127, -0.13277852346573402], [-0.13294465237215997, -0.1331343744731282, -0.13315537746712325, -0.13297264620540483, -0.13297221070219528, -0.1331608555788659, -0.1337974354021675, -0.13366029282378541, -0.13397829019364643, -0.13347118333006328, -0.13380547261304465, -0.13415791553132203, -0.13436743143778923, -0.13416465137955633, -0.1336944626800391, -0.13391189855159902, -0.13350966407890932, -0.13366670150662655, -0.13368039256028455, -0.13347009962509598], [-0.133376600865105, -0.13395481344944193, -0.1339955846830665, -0.133956967884642, -0.13444739915933085, -0.13480443484205623, -0.13553775345604469, -0.13577815788119485, -0.13626241644698478, -0.13578778100304814, -0.13600939090830583, -0.13605401743367845, -0.1363863505755896, -0.13632887707726826, -0.13590477361164166, -0.13548728900052692, -0.13504306343454786, -0.13434553140256977, -0.134204688920121, -0.13377243388378493], [-0.1336682588237614, -0.13422447217878333, -0.13491126661397695, -0.13489108653969023, -0.1356255820450017, -0.13641858768724696, -0.13726032358608364, -0.13756147425761883, -0.13826732839332784, -0.13787068229003774, -0.13819141478504252, -0.13814020164934854, -0.1383025679443424, -0.13767489897776403, -0.1370517969258808, -0.13651091961430573, -0.13533791682069152, -0.13495068828901735, -0.13448202290108713, -0.13383517463969868], [-0.13388448192593644, -0.13452246644280663, -0.1348825936438942, -0.13548641134956727, -0.13607722308562042, -0.1369913125177349, -0.13804634592340168, -0.1385997471309521, -0.1393396940160915, -0.13934838346032416, -0.13920885511607672, -0.13948125985373397, -0.13893318047380865, -0.1379397712645341, -0.13715709296524092, -0.13626258823899745, -0.1353994598816213, -0.1347628519489198, -0.1342948953293206, -0.1338826651952545], [-0.13396856227055137, -0.13388308324032946, -0.1349033619784188, -0.13485684121421254, -0.1358148424531872, -0.1365104818532411, -0.13741175304944797, -0.13811134914899487, -0.13850002869344977, -0.13841450536318534, -0.13862883436250045, -0.13852386431366803, -0.13818160725162842, -0.1369681240039362, -0.1362562280554694, -0.13548377081345972, -0.13483066956948572, -0.13443735012047295, -0.1342378731397958, -0.13377307509823724], [-0.13356343572314888, -0.1341941365836396, -0.1342048717962691, -0.13437430888148577, -0.13448523278647978, -0.13473340434566053, -0.13563618405175148, -0.13570696814363353, -0.13620209549575168, -0.13629332827180524, -0.1360534850897276, -0.13616043752292084, -0.13581500811714792, -0.13516798139559938, -0.13479299366693354, -0.1341684228711022, -0.13401951858470776, -0.13409658215468903, -0.13379318780279842, -0.13390389491094368], [-0.1333330167529305, -0.13362161369838121, -0.1338481709725886, -0.1338547076999006, -0.13402849942936956, -0.13371246447901386, -0.13406075991101218, -0.1346068155255807, -0.13448339135153925, -0.1343697655445329, -0.13433244392480195, -0.1347059206824048, -0.13430621020656403, -0.13398494532138386, -0.13408981243260248, -0.1339676492377287, -0.13363640585529052, -0.133463268599468, -0.1337636217634856, -0.13313319646196237], [-0.13339001677501267, -0.13356763117486625, -0.1335138731471422, -0.13369904065728763, -0.13356265784698806, -0.13393646575303964, -0.13379523451932357, -0.13422171713427905, -0.13424327801179983, -0.13430096809440317, -0.1340738456131889, -0.13400142245434493, -0.13425066634473476, -0.13324811503065892, -0.13383708673162248, -0.13367917914076613, -0.13306466082536614, -0.13363437140568288, -0.13351391502054588, -0.13366421283666058], [-0.13340084146025155, -0.13360379024948849, -0.1331487959310442, -0.13371310305092954, -0.13353330390356052, -0.13374704532881462, -0.1339920647140691, -0.13400128635678848, -0.13403768677352734, -0.1340789146755405, -0.1338463733795615, -0.13397139870497204, -0.13388109750858204, -0.1338416154765018, -0.13375936615743866, -0.1334771725677485, -0.13331791869274598, -0.13357071928634118, -0.13323267315952836, -0.1336530524531351], [-0.1332864922744885, -0.13355810189570258, -0.1333536633933724, -0.13342457051287818, -0.13360138120726672, -0.13342527909246157, -0.13348951207010357, -0.13395044891119165, -0.13383389597868128, -0.1338742842122126, -0.13356563240167563, -0.13390620276042048, -0.13383512262365405, -0.13344925360869556, -0.13366710661155234, -0.1334383076256932, -0.13325524216196766, -0.13304944832786095, -0.13323367495327598, -0.13339053344025073]]
  in  "Channel":i32=4
  in  "Abort MCL Scan":bool
  out "MCL Scan I":u64=2
  out "MCL Scanning":bool
  in  "Start MCL Scan":bool
  out "wait to reset values":bool
  in  "Tab Control 4":enum32{"Scan Settings", "MCL FPGA Loop Timing"}(tab)
  out "Total Time (s)":dbl=48.0
  in  "Scan lines (y)":u64=20
  in  "Fast Scan Dir":bool=TRUE
  in  "2D or 1D Scan":bool=TRUE
  out "Initial X":dbl=1.0296389660328993
  out "Initial Y":dbl=4.906247662064187
  out "Time/f+b scan (s) (MCL)":dbl=2.4 caption="Time/scan (s)"
  in  "Number of scans (MCL)":u64=1 caption="Scans"
  in  "Scan steps (MCL)":u64=40 caption="Scan steps (x)"
  in  "N APD Samp/step":dbl=3.0
  in  "Scan Range (V)\n(of steps)":dbl=3.5
  in  "Restart DMA? (MCL)":bool=TRUE caption="Restart DMA?"
  in  "Continuous MCL Scanning":bool caption="Cont. Scanning"
  in  "Center Scan":bool=TRUE
  in  "Save Data (MCL)":bool=TRUE caption="Save Data"
  out "Actual Incr. int (MCL)":i16=294 caption="Incr. int"
  out "Desired incr (int)":dbl=294.0628205128205
  out "Desired Scan Incr (V)":dbl=0.08974358974358974
  out "N sets should be saved (MCL)":dbl=160.0 caption="N sets should be saved"
  out "Data points/scans (MCL)":dbl=4800.0 caption="Data points/scans"
  out "Data points/scan (f+b)":dbl=240.0 caption="points/scan (f+b)"
  out "Cycles/step (MCL)":u64=2000 caption="Cycles/step" format="%.0p"
  out "Actual MCL Inc (V)":dbl=0.08972441785943175
  in  "Phase adjust (MCL)":i16 caption="Phase adjust"
  out "Relative Phase (MCL)":i16 caption="Relative Phase"
  in  "Initial Phase Adj. (MCL)":i16 caption="Initial Phase Adj."
  in  "Update Count (MCL)":u32=600
  in  "+ phase (MCL)":bool
  in  "- phase (MCL)":bool
  out "MCL Late Counter":u32
  in  "APD 1 AO Mult.":i16=1 min=1
  in  "APD 2 AO Mult.":i16=1 min=1
  in  "Tab Control 7":enum32{"Green FB Signals", "Slow MCL Scan"}(tab)
  out "Green FB Plot":dbl(graph)=-0.013428144169438765
  out "MCL Scan 2":cluster{"Begin (V)":dbl, dbl, dbl[]}(graph)
  out "MCL Scan":cluster{"Begin (V)":dbl, dbl, dbl[]}(graph)
  in  "Green laser mode":enum32{"Laser ON", "Laser OFF", "Interlace"}(radio)=enum."Interlace"
  in  "GI Frequency, ON count":u32=150 min=1 step=1
  in  "Invert GI":bool
  out "GI Late Counter":u32
  in  "Phase adj. (GI)":i16=5
  out "GI relative phase":i16
  in  "+ phase (GI)":bool
  in  "Initial Phase Adjustment (GI)":i16=19
  in  "GI Frequency, OFF count":u32=450 min=1 step=1
  in  "- phase (GI)":bool
  out "Green FB Signals (V)":cluster{"Y":dbl, "X":dbl, "Sum":dbl}={"Y"=-744.7045454545455, "X"=-744.7045454545455, "Sum"=-0.013428144169438765}
  out "Relative phase (Green FB)":i16
  in  "+ phase (Green FB)":bool
  in  "- phase (Green FB)":bool
  in  "Green FB Count":u32=600
  in  "Phase adj. (Green FB)":i16=10
  in  "Initial Phase Adjustment (Green FB)":i16=50
  in  "Green FB On/Off":bool=TRUE
  in  "Current When FB OFF (%)":dbl=87.0 min=0.0 max=100.0 step=1.0
  in  "Green int current ON count adj":u32=150
  in  "Green FB Gains":T14={"proportional gain (Kc)"=10, "integral gain (Kc*Ts/Ti)"=5, "derivative gain (Kc*Td/Ts)"=0}
  in  "Green FB Setpoint (mV)":dbl=100.0
  in  "- phase (GI) 2":bool
  in  "Initial Phase Adjustment (GI) 2":i16=-100
  in  "+ phase (GI) 2":bool
  out "GI relative phase 2":i16
  in  "Phase adj. (GI) 2":i16=20
  out "GI Late Counter 2":u32
  in  "Trap Position FIFO Depth":u32=300000 format="%.0p"
  in  "# Samples/trap":u32=20000 format="%.0p"
  out "Trap AI Elements/DMA read":u32=320000 format="%.0p"
  out "Ave. Rate (Hz)":dbl=200000.0 format="%#_6p"
  out "FIFO El. Rem.":u32 format="%.0p"
  in  "Phase adj. (AI1)":i16=15
  out "Relative phase (AI1)":i16
  in  "+ phase (AI1)":bool
  in  "- phase (AI1)":bool
  out "Late Counter (AI1)":u32
  in  "Initial Phase Adjustment (AI1)":i16=220
  out "AI rate (Hz)":dbl=200000.0 format="%#_6p"
  in  "AI Count (ticks)":u32=200
  out "# Samples/channel":u32=40000 format="%.0p"
  in  "Trap AI FIFO Depth":u32=600000 format="%.0p"
  in  "Detector Type":string(combo)="IR-QPD + PSD + FB-QPD X position"
  in  "N Acq Sets (Traps + Fl.)":i16=3
  in  "Sets to FIFO (Traps)":T15={"Set 1"=TRUE, "Set 2"=TRUE, "Set 3"=FALSE}
  in  "FPGA Ave.":dbl=1.0 min=1.0 step=1.0
  out "Ave. Period (s)":dbl=5e-06 format="%#_6p"
  out "DMA Update Period (s)":dbl=0.3
  out "FPGA Averaging":bool
  out "Trap Sets":u32=2
  out "Counts/DMA":dbl=12000000.0 format="%#_6p"
  out "Trap Pos FIFO El Remaining":u32=306
  out "Trap Pos Elements/DMA read":u32=120000 format="%.0p"
  out "Trap AI FIFO Timeout":u16
  out "Trap Pos FIFO Timeout":u16
  in  "Video Capture Rate (Hz)":dbl=30.0
  in  "Video Index":dbl=1.0 min=1.0 step=1.0
  in  "New Video File":bool
  in  "Save Video":bool
  in  "Reset Averaging":bool
  in  "Averaging":bool
  in  "Save Image":bool
  in  "Image Index":dbl=1.0 min=1.0
  out "Path Out":path
  in  "Center Point":cluster{"X":i32, "Y":i32}={"X"=335, "Y"=271}
  in  "Zoom Factor":sgl=7.0
  out "Window Size":cluster{"Width":i32, "Height":i32}
  out "Window Position":cluster{"X Position":i32, "Y Position":i32}={"X Position"=40, "Y Position"=40}
  in  "Initial Window Size":cluster{"Width":i32, "Height":i32}={"Width"=884, "Height"=619}
  in  "Initial Window Position":cluster{"X Position":i32, "Y Position":i32}={"X Position"=796, "Y Position"=4}
  in  "Intensity Upper":dbl=88.0
  in  "Intensity Lower":dbl=66.0
  out "error out":errorcluster
  out "error out 2":errorcluster
  in  "Harvard Syringe Pump Serial Port":refnum<visa-resource-name>="ASRL5::INSTR"
  in  "Lost Tether Alarm Threshold (pN)":dbl=0.5
  in  "AOM X Cal (nm/MHz)":dbl=123.0
  in  "MCL X Cal (nm/V)":dbl=1070.0
  out "X RF Amplitude Limits (%)":T16={"Minimum"=0.0, "Maximum"=50.0, "Increment"=1.0}
  out "X RF Frequency Limits (MHz)":T16={"Minimum"=60.0, "Maximum"=90.0, "Increment"=1.0}
  out "Y RF Frequency Limits (MHz)":T16={"Minimum"=0.0, "Maximum"=40.0, "Increment"=1.0}
  out "Y RF Amplitude Limits (%)":T16={"Minimum"=0.0, "Maximum"=50.0, "Increment"=1.0}
  in  "Manip. X?":bool=TRUE
  in  "Manip. Y?":bool
  in  "Force Manip Abort":bool
  out "Read cal error":errorcluster
  in  "DAQ Delay (ms)":u32=1000
  in  "Start Scan":bool
  in  "Scan axis":bool=TRUE
  in  "Osc. amp. (V)":dbl=5.0
  in  "Osc. center (V)":dbl=5.0
  in  "Osc. freq. (Hz) 2":dbl=1.0
  in  "MCL Mode":u16(ring) items=["Manual Positioning", "Sinusoidal Wave", "Linear Scan"]
  in  "Begin (V)":dbl
  in  "End (V)":dbl=10.0
  in  "N Points":dbl=20.0
  in  "Delay to Interlace (s)":dbl
  in  "Delayed Interlace Start":bool
  in  "Read Lateness and Rel Phase":bool
  out "Vec Mean of T1 T2":dbl[](array[numeric])=[107.52745637613502, 108.18516687787962]
  in  "Cal read wait (s)":u32=5
  out "Time tether formed":timestamp=timestamp(3374779860.98425 s since 1904-01-01)
  in  "Sample Chamber Stage Serial Port":refnum<visa-resource-name>="ASRL4::INSTR"
  in  "Chemyx Syringe Pump Serial Port":refnum<visa-resource-name>="ASRL3::INSTR"
  in  "Limit Min (MHz)":dbl=10.0 caption="Min (MHz)"
  in  "Limit Max (MHz)":dbl=16.0 caption="Max (MHz)"
  in  "Limits Enable":bool=TRUE caption="Enable"
  out "AI labels":string[](array[string])=["T1 Y", "T1 X", "T1 Sum", "T2 Y", "T2 X", "T2 Sum", "T1 FB X", "T1 FB Sum", "T2 FB X", "T2 FB Sum", "PSD Y", "PSD X", "PSD Y Sum"]
  in  "Save Trap Pos. Data":bool=TRUE
  # "After"
  # "During"
  # "Trap On?"
  # "BD Flow ON?"
  # "Samp Flow ON?"
  # "1"
  # "2"
  # "Trap Display:"
  # "APD Display:"
  # "DAQ"
  # "Trap Manipulation"
  # "Data Saving"
  # "Bead Calibration"
  # "Harvard Pump\n(sample channel for flow exp)"
  # "Chemyx Pump 2"
  # "Units: \n1 = ml/m\n2 = ml/h\n3 = ul/m\n4 = ul/h"
  # "Rate param is ul/h\nVolume param is ul"
  # "X"
  # "Y"
  # "Oscillate Set 1 freq. (debugging)"
  # "BD 1"
  # "BD 2"
  # "AOD Raster Scan"
  # "Approx. trap separations"
  # "X"
  # "Y"
  # "FPGA\nreading"
  # "DMA\ntransfer"
  # "APD Gates"
  # "APD 2"
  # "APD 1"
  # "X"
  # "2D"
  # "Y"
  # "1D"
  # "Green Laser Interlacing"
  # "Green FB Measurement"
  # "Digital Gate"
  # "Current Analog Control"
  # "Total AI Rates (NOT rates/trap)"
  # "(Samples/trap x Trap Sets)"
  # "(Samples/channel x\n8 if averaging (8 channels)\n4 if no averaging)"
  # "Trap 1"
  # "Trap 2"
  # "Flour./Trap 3"
  # "External Video Window"
  # "MCL Position Debugging"
  # "Temporary Control Storage\n(these used to be somewhere else, still want to keep them)"
  # "Y"
  # "X"
  # "Trap Position Difference Limits"